vi "MPS_main.vi"() -> ()   [LabVIEW 2021] (continued)
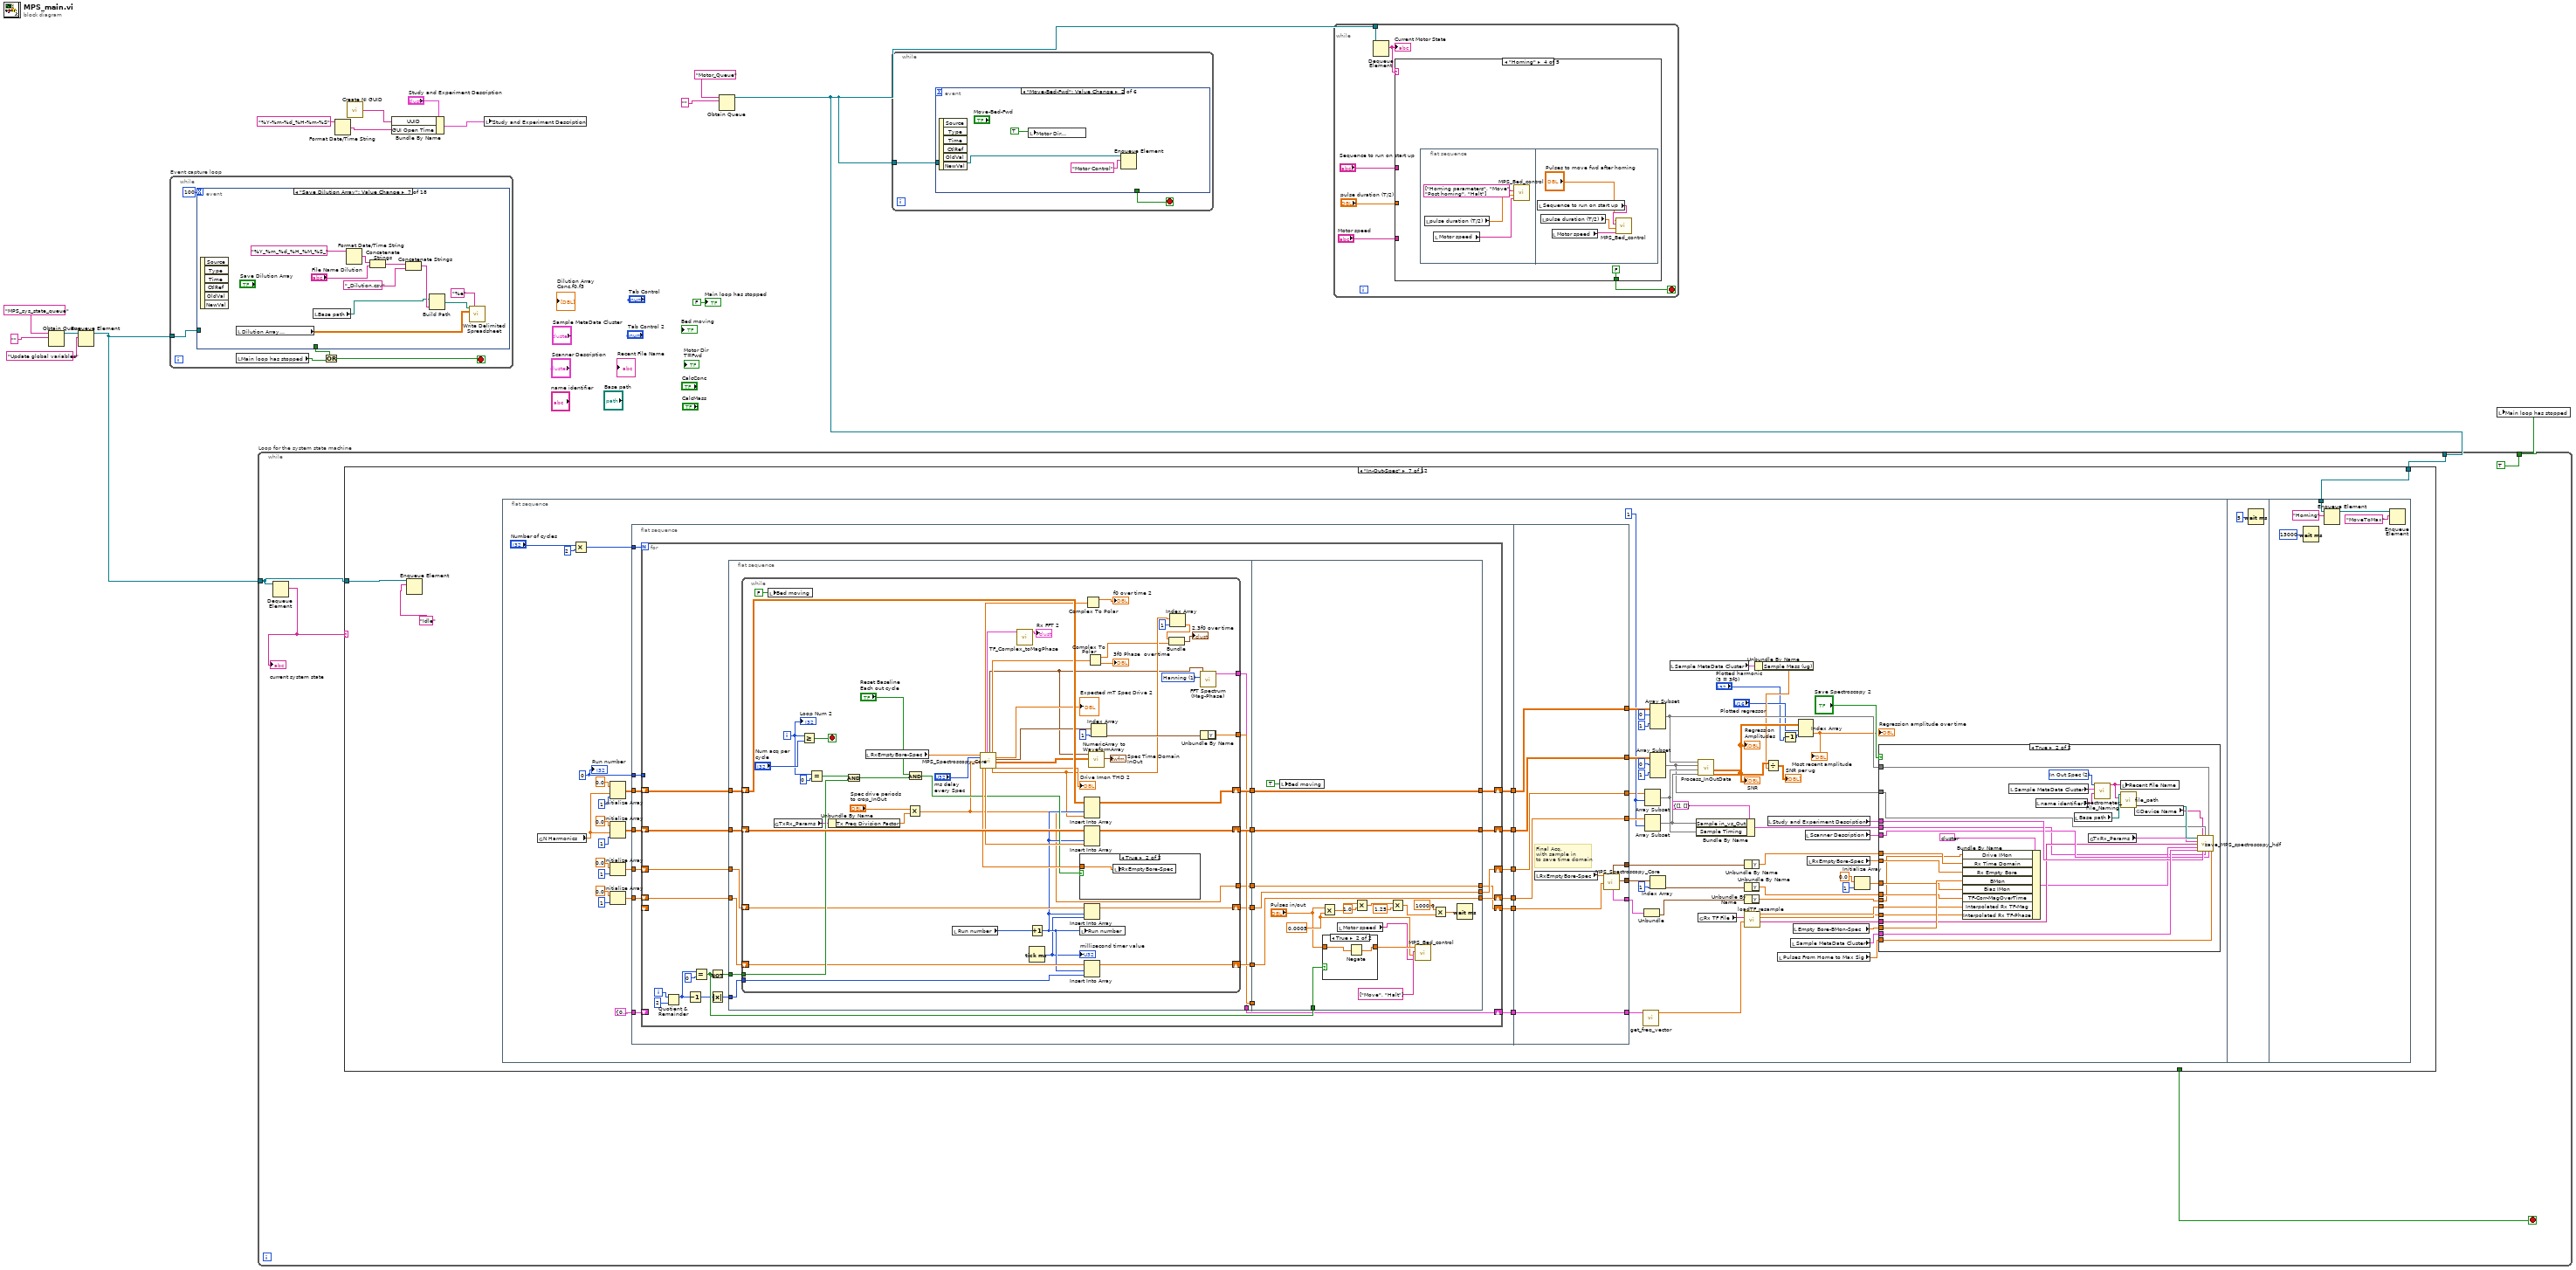
[diagram p0: block diagram]
diagram:
  n1 = Obtain Queue(name (unnamed)="MPS_sys_state_queue", element data type="") -> (queue out=w11:refnum<queue>)  [unwired: 3 in, 2 out]
  n2 = Enqueue Element(queue=w11, element="Update global variables") -> (queue out=w9:refnum<queue>)  [unwired: 2 in, 2 out]
  n3 = while "Event capture loop" {
    tunnel: w9 -> [w19]
    stop <- w16 stop-if-true
    n4 = event shown="[6] \"Save Dilution Array\": Value Change" {
      selector: _ -> [_ _ _ _ _ _ _ _ _ _ _ _ _ _ _ _ _ _]
      dyn-events: _ -> [_ _ _ _ _ _ _ _ _ _ _ _ _ _ _ _ _ _]
      timeout: 100 -> [_ _ _ _ _ _ _ _ _ _ _ _ _ _ _ _ _ _]
      tunnel: w19 -> [_ w22 _ w31 w33 _ _ _ w74 w78 w80 w82 w84 _ _ _ w105 w108]
      tunnel: [FALSE ("x") _ _ _ _ _ _ _ _ _ _ _ _ _ _ _ _ TRUE ("x")] -> w17
      event Timeout {
        n5 = event-data() -> ()  [unwired: 1 in, 3 out]
      }
      event "Run Sys Ref Meas": Value Change {
        n6 = event-data() -> ()  [unwired: 1 in, 6 out]
        n7 = Enqueue Element(queue=w22, element="System Reference Measurement") -> ()  [unwired: 2 in, 3 out]
      }
      event "Divide Mass by X": Value Change {
        n8 = event-data() -> ()  [unwired: 1 in, 6 out]
        n9 = local read "Sample MetaData Cluster"() -> (w29:T1)
        n10 = Unbundle By Name(w29) -> ("Sample Mass (ug)"=w30:dbl, "Sample Conc(mg/mL)"=w26:dbl)
        n11 = Divide(x=w30, y="Divide By val") -> (x/y=w27:dbl)
        n12 = Divide(x=w26, y="Divide By val") -> (x/y=w24:dbl)
        n13 = Bundle By Name(cluster=w29, "Sample Mass (ug)"=w27, "Sample Conc(mg/mL)"=w24) -> (w28:T1)
        n14 = local write "Sample MetaData Cluster"(w28) -> ()
      }
      event "Run Spectroscopy": Value Change {
        n15 = event-data() -> ()  [unwired: 1 in, 6 out]
        n16 = Enqueue Element(queue=w31, element="Spectroscopy") -> ()  [unwired: 2 in, 3 out]
      }
      event "Run DilutionAdd": Value Change {
        n17 = event-data() -> ()  [unwired: 1 in, 6 out]
        n18 = Enqueue Element(queue=w33, element="Acquire Dilution Data") -> ()  [unwired: 2 in, 3 out]
      }
      event "Clear Dilution Array": Value Change {
        n19 = event-data() -> ()  [unwired: 1 in, 6 out]
        n20 = Initialize Array(0.0 ("element"), 0 ("dimension size"), 3 ("dimension size")) -> (w35:dbl[][])
        n21 = local write "Dilution Array\nConc,f0,f3"(w35) -> ()
        n22 = Index Array(array=w35, index (col)=0 ("disabled index (col)")) -> (element=w42:dbl[])  [unwired: 1 in]
        n23 = Index Array(array=w35, index (col)=2 ("disabled index (col)")) -> (element=w43:dbl[])  [unwired: 1 in]
        n24 = call <vilib>:"Linear Fit.vi"("Y"=w43, "X"=w42) -> ("Best Linear Fit"=w41:dbl[])  [unwired: 9 in, 4 out]
        n25 = Bundle(w42, w43) -> (w39:cluster{dbl[], dbl[]})  [unwired: 1 in]
        n26 = call <vilib>:"Correlation Coefficient (Spearman).vi"("Y"=w43, "X"=w42) -> ()  [unwired: 8 in, 2 out]
        n27 = Bundle(w42, "Best Linear Fit"=w41) -> (w40:cluster{dbl[], "Best Linear Fit":dbl[]})  [unwired: 1 in]
        n28 = Build Array(w40, w39) -> (w38:cluster{dbl[], "Best Linear Fit":dbl[]}[])
        n29 = local write "3f0 vs Mass"(w38) -> ()
      }
      event "Save Dilution Array": Value Change {
        n30 = event-data() -> ()  [unwired: 1 in, 6 out]
        n31 = local read "Dilution Array\nConc,f0,f3"() -> (w49:dbl[][])
        n32 = local read "Base path"() -> (w47:path)
        n33 = Format Date/Time String(time format string (%c)="%Y_%m_%d_%H_%M_%S_") -> (date/time string=w54:string)  [unwired: 2 in]
        n34 = Concatenate Strings(w54, "File Name Dilution") -> (w56:string)
        n35 = Concatenate Strings(w56, "_Dilution.csv" ("string")) -> (w55:string)
        n36 = Build Path(base path=w47, name or relative path=w55) -> (appended path=w50:path)
        n37 = call-poly <vilib>:"Write Delimited Spreadsheet.vi"("file path (dialog if empty)"=w50, "format (%.3f)"="%e", "2D data"=w49) -> ()  [unwired: 11 in, 2 out]
      }
      event "Delete Last Meas": Value Change {
        n38 = event-data() -> ()  [unwired: 1 in, 6 out]
        n39 = local read "Dilution Array\nConc,f0,f3"() -> (w72:dbl[][])
        n40 = Array Size(array=w72) -> (size(s)=w71:i32[])
        n41 = Index Array(array=w71, index=0) -> (element=w69:i32)
        n42 = Decrement(x=w69) -> (x-1=w68:i32)
        n43 = Array Subset(array=w72, index (row)=0 ("index"), length (row)=w68, index (col)=0 ("index")) -> (w58:dbl[][])  [unwired: 1 in]
        n44 = local write "Dilution Array\nConc,f0,f3"(w58) -> ()
        n45 = Index Array(array=w58, index (col)=0 ("disabled index (col)")) -> (element=w64:dbl[])  [unwired: 1 in]
        n46 = Index Array(array=w58, index (col)=2 ("disabled index (col)")) -> (element=w65:dbl[])  [unwired: 1 in]
        n47 = call <vilib>:"Linear Fit.vi"("Y"=w65, "X"=w64) -> ("Best Linear Fit"=w63:dbl[])  [unwired: 9 in, 4 out]
        n48 = Bundle(w64, w65) -> (w61:cluster{dbl[], dbl[]})  [unwired: 1 in]
        n49 = call <vilib>:"Correlation Coefficient (Spearman).vi"("Y"=w65, "X"=w64) -> ()  [unwired: 8 in, 2 out]
        n50 = Bundle(w64, "Best Linear Fit"=w63) -> (w62:cluster{dbl[], "Best Linear Fit":dbl[]})  [unwired: 1 in]
        n51 = Build Array(w62, w61) -> (w57:cluster{dbl[], "Best Linear Fit":dbl[]}[])
        n52 = local write "3f0 vs Mass"(w57) -> ()
      }
      event "Run in-out spec": Value Change {
        n53 = event-data() -> ()  [unwired: 1 in, 6 out]
        n54 = for {
          N: "Number of \nsaved runs" -> [_]
          tunnel: w74 -> [w75]
          n55 = flat-sequence {
            tunnel: w75 -> [w76]
            frame #0 {
              n56 = Enqueue Element(queue=w76, element="In-Out-Spec") -> ()  [unwired: 2 in, 3 out]
            }
            frame #1 {
            }
          }
        }
      }
      event "Run Mag": Value Change {
        n57 = event-data() -> ()  [unwired: 1 in, 6 out]
        n58 = Enqueue Element(queue=w78, element="Magnetometry") -> ()  [unwired: 2 in, 3 out]
      }
      event "Acq Baseline": Value Change {
        n59 = event-data() -> ()  [unwired: 1 in, 6 out]
        n60 = Enqueue Element(queue=w80, element="Acquire Empty Bore") -> ()  [unwired: 2 in, 3 out]
      }
      event "Zero Baseline": Value Change {
        n61 = event-data() -> ()  [unwired: 1 in, 6 out]
        n62 = Enqueue Element(queue=w82, element="Zero Baseline") -> ()  [unwired: 2 in, 3 out]
      }
      event "Run Cal BMon": Value Change {
        n63 = event-data() -> ()  [unwired: 1 in, 6 out]
        n64 = Enqueue Element(queue=w84, element="Cal_BMon") -> ()  [unwired: 2 in, 3 out]
      }
      event "CalcMass": Value Change {
        n65 = event-data() -> ()  [unwired: 1 in, 6 out]
        n66 = local read "Sample MetaData Cluster"() -> (w90:T1)
        n67 = Unbundle By Name(w90) -> ("Sample Volume (uL)"=w89:dbl, "Sample Conc(mg/mL)"=w88:dbl)
        n68 = Multiply(x=w89, y=w88) -> (x*y=w86:dbl)
        n69 = Bundle By Name(cluster=w90, "Sample Mass (ug)"=w86) -> (w87:T1)
        n70 = local write "Sample MetaData Cluster"(w87) -> ()
      }
      event "CalcConc": Value Change {
        n71 = event-data() -> ()  [unwired: 1 in, 6 out]
        n72 = local read "Sample MetaData Cluster"() -> (w95:T1)
        n73 = Unbundle By Name(w95) -> ("Sample Mass (ug)"=w94:dbl, "Sample Volume (uL)"=w93:dbl)
        n74 = Divide(x=w94, y=w93) -> (x/y=w91:dbl)
        n75 = Bundle By Name(cluster=w95, "Sample Conc(mg/mL)"=w91) -> (w92:T1)
        n76 = local write "Sample MetaData Cluster"(w92) -> ()
      }
      event "Toggle fan": Value Change {
        n77 = event-data() -> ()  [unwired: 1 in, 6 out]
        n78 = global read "MPS_global_variables.vi" "Fan Control Line"() -> (w100:tag)
        n79 = call-poly <vilib>:"DAQmx Create Virtual Channel.vi"("lines"=w100) -> ("task out"=w102:refnum<k21>, "error out"=w103:errorcluster)  [unwired: 13 in]
        n80 = call-poly <vilib>:"DAQmx Write.vi"("task/channels in"=w102, "data"="Toggle fan", "error in"=w103) -> ("task out"=w99:refnum<k21>, "error out"=w98:errorcluster)  [unwired: 10 in, 1 out]
        n81 = call <vilib>:"DAQmx Stop Task.vi"("task/channels in"=w99, "error in"=w98) -> ("task out"=w97:refnum<k21>, "error out"=w96:errorcluster)  [unwired: 12 in]
        n82 = call <vilib>:"DAQmx Clear Task.vi"("task in"=w97, "error in"=w96) -> ()  [unwired: 13 in, 1 out]
      }
      event "Update global variables Button": Value Change {
        n83 = event-data() -> ()  [unwired: 1 in, 6 out]
        n84 = Enqueue Element(queue=w105, element="Update global variables") -> ()  [unwired: 2 in, 3 out]
      }
      event "stop": Value Change {
        n85 = event-data() -> ()  [unwired: 1 in, 6 out]
        n86 = Enqueue Element(queue=w108, element="Halt") -> ()  [unwired: 2 in, 3 out]
      }
    }
    n87 = local read "Main loop has stopped"() -> (w18:bool)
    n88 = Or(x=w17, y=w18) -> (x .or. y?=w16:bool)
  }
  n89 = Format Date/Time String(time format string (%c)="%Y-%m-%d_%H-%m-%S") -> (date/time string=w4:string)  [unwired: 2 in]
  n90 = call <vilib>:"Create NI GUID.vi"() -> ("NI GUID"=w7:string)
  n91 = Bundle By Name(cluster="Study and Experiment Description", "UUID"=w7, "GUI Open Time"=w4) -> (w6:T5)
  n92 = local write "Study and Experiment Description"(w6) -> ()
  n93 = Obtain Queue(name (unnamed)="Motor_Queue", element data type="") -> (queue out=w1:refnum<queue>)  [unwired: 3 in, 2 out]
  n94 = while "Loop for the system state machine" {
    tunnel: w9 -> [w111]
    tunnel: [TRUE ("Main loop has stopped")] -> w12
    tunnel: w1 -> [w109]
    stop <- w113 stop-if-true
    n95 = Dequeue Element(queue=w111) -> (element=w110:string)  [unwired: 2 in, 3 out]
    "current system state" <- w110
    n96 = case shown="\"In-Out-Spec\"" w110 {
      tunnel: [_ _ _ _ _ _ _ _ _ _ _ TRUE] -> w113
      tunnel: w111 -> [_ w116 w187 w335 w388 w532 w546 _ w820 w917 w981 _]
      tunnel: w109 -> [_ _ _ _ _ _ w545 _ _ _ _ _]
      frame "Idle", Default {
      }
      frame "Update global variables" {
        n97 = Enqueue Element(queue=w116, element="Idle") -> ()  [unwired: 2 in, 3 out]
        n98 = flat-sequence {
          tunnel: [w124] -> w114
          tunnel: w114 -> [w132]
          frame #0 {
            n99 = Unbundle By Name("TxRx_Params") -> ("sample rate"=w128:dbl, "Tx Freq Division Factor"=w126:dbl, "Drive Periods per Bias"=w125:dbl)
            n100 = global read "MPS_global_variables.vi" "N Harmonics"() -> (w120:dbl)
            n101 = Subtract(x=w120, y=2.0) -> (x-y=w121:dbl)
            n102 = Divide(x=w128, y=w126) -> (x/y=w123:dbl)
            n103 = for {
              N: w121 -> [_]
              tunnel: [w130] -> w118 mode=indexing
              i -> [w131]
              n104 = Add(x=w131, y=2) -> (x+y=w130:i32)
            }
            n105 = Divide(x=w123, y=w125) -> (x/y=w127:dbl)
            n106 = Multiply(x=w123, y=w118) -> (x*y=w117:dbl[])
            n107 = Bundle By Name(cluster="TxRx_Params", "Tx freq"=w123, "Bias freq"=w127, "TX harmonics"=w117) -> (w124:T2)
            n108 = global write "MPS_global_variables.vi" "TxRx_Params"(w124) -> ()
          }
          frame #1 {
            n109 = local write "TxRx_Params"(w132) -> ()
          }
        }
      }
      frame "System Reference Measurement" {
        w146 = dbl[][] [] ("array")
        n110 = Enqueue Element(queue=w187, element="Idle") -> ()  [unwired: 2 in, 3 out]
        n111 = global read "MPS_global_variables.vi" "N Harmonics"() -> (w133:dbl)
        n112 = Initialize Array(0.0 ("element"), w133, 0 ("dimension size")) -> (w184:dbl[][])
        n113 = Initialize Array(0.0 ("element"), w133, 0 ("dimension size")) -> (w181:dbl[][])
        n114 = for {
          N: "Num Avgs SRM" -> [_]
          tunnel: "Num Avgs SRM" -> [_]
          shift-right: [w254] -> w151
          shift-left: w184 -> [w284]
          shift-right: [w253] -> w160
          shift-left: w181 -> [w283]
          shift-right: [w273] -> _
          shift-left: w146 -> [w280]
          shift-right: [w272] -> _
          shift-left: w146 -> [w277]
          shift-right: [w247] -> _
          shift-left: w146 -> [w274]
          shift-right: [w261] -> _
          shift-left: w146 -> [w271]
          shift-right: [w263] -> _
          shift-left: w146 -> [w270]
          shift-right: [w232] -> w145
          shift-left: _ -> [_]
          tunnel: [w228] -> w136
          i -> [w282]
          # "Rx FFT"
          # "PSD"
          # "Tx FFT"
          n115 = global read "MPS_global_variables.vi" "TxRx_Params"() -> (w289:T2)
          n116 = global read "MPS_global_variables.vi" "TxRx_Params"() -> (w255:T2)
          n117 = local read "RxEmptyBore-Spec"() -> (w291:dbl[])
          n118 = Unbundle By Name(w289) -> ("Tx Freq Division Factor"=w288:dbl)
          n119 = Multiply(x="Spec Tx periods\nto crop SRM", y=w288) -> (x*y=w227:dbl)
          n120 = Unbundle By Name(w255) -> ("TX harmonics"=w242:dbl[], "Tx freq"=w240:dbl)
          n121 = call "MPS_Spectroscopy_Core.vi"("EmptyBoreBaseline_Spec"=w291, "ms delay"="ms delay SRM", "Spec samples\nto crop"=w227) -> ("phase f1-f9"=w281:dbl[], "TF Corr Rx FFT complex"=w279:T12, "TF units from loaded file"=w228:string, "TxIMon cluster"=w222:T13, "mag f1-f9"=w285:dbl[])  [unwired: 2 in, 10 out]
          n122 = Unbundle(w222) -> ("TF Corr Rx FFT complex"=w221:T12)  [unwired: 1 out]
          n123 = call "TF_Complex_toMagPhase.vi"("TF Corr Rx FFT Mag"=w221) -> ("phase"=w268:dbl[], "magnitude"=w269:dbl[])  [unwired: 4 in, 5 out]
          n124 = call "TF_Complex_toMagPhase.vi"("TF Corr Rx FFT Mag"=w279) -> ("phase"=w276:dbl[], "magnitude"=w278:dbl[], "Freq array"=w220:dbl[], "PSD"=w275:dbl[])  [unwired: 4 in, 3 out]
          n125 = Equal?(x=0, y=w282) -> ()  [unwired: 1 out]
          n126 = Insert Into Array(array=w274, new element=w275) -> (w247:dbl[][])  [unwired: 2 in]
          n127 = Insert Into Array(array=w277, new element=w276) -> (w272:dbl[][])  [unwired: 2 in]
          n128 = Insert Into Array(array=w271, new element=w269) -> (w261:dbl[][])  [unwired: 2 in]
          n129 = Insert Into Array(array=w270, new element=w268) -> (w263:dbl[][])  [unwired: 2 in]
          n130 = Insert Into Array(array=w280, new element=w278) -> (w273:dbl[][])  [unwired: 2 in]
          n131 = Insert Into Array(array=w284, index (col)=w282, new element=w285) -> (w254:dbl[][])  [unwired: 1 in]
          n132 = Insert Into Array(array=w283, index (col)=w282, new element=w281) -> (w253:dbl[][])  [unwired: 1 in]
          n133 = Insert Into Array(array=w242, index=0, new element=w240) -> (w239:dbl[])
          n134 = Polar To Complex(1:w263, 2:w261) -> (0:w262:cdb[][])
          n135 = Polar To Complex(1:w272, 2:w273) -> (0:w267:cdb[][])
          n136 = Polar To Complex(1:w253, 2:w254) -> (0:w245:cdb[][])
          n137 = Transpose 2D Array(2D array=w262) -> (transposed array=w264:cdb[][])
          n138 = Transpose 2D Array(2D array=w267) -> (transposed array=w266:cdb[][])
          n139 = Transpose 2D Array(2D array=w247) -> (transposed array=w265:dbl[][])
          n140 = for {
            tunnel: w245 -> [w295] mode=indexing
            tunnel: [w294] -> w244 mode=indexing
            tunnel: [w292] -> w243 mode=indexing
            n141 = call "mean_std_var_Complex.vi"("Input Array"=w295) -> ("standard deviation"=w294:dbl, "mean"=w293:cdb)  [unwired: 8 in, 1 out]
            n142 = Complex To Polar(r * e^(i*theta)=w293) -> (r=w292:dbl)  [unwired: 1 out]
          }
          n143 = for {
            tunnel: w265 -> [w302] mode=indexing
            tunnel: [w304] -> w231 mode=indexing
            tunnel: [w303] -> w230 mode=indexing
            tunnel: w266 -> [w301] mode=indexing
            tunnel: [w300] -> w238 mode=indexing
            tunnel: [w299] -> w229 mode=indexing
            tunnel: w264 -> [w298] mode=indexing
            tunnel: [w297] -> w237 mode=indexing
            tunnel: [w296] -> w233 mode=indexing
            n144 = call "mean_std_var_Complex.vi"("Input Array"=w301) -> ("standard deviation"=w299:dbl, "mean"=w300:cdb)  [unwired: 8 in, 1 out]
            n145 = call "mean_std_var_Complex.vi"("Input Array"=w302) -> ("standard deviation"=w303:dbl, "mean"=w304:cdb)  [unwired: 8 in, 1 out]
            n146 = call "mean_std_var_Complex.vi"("Input Array"=w298) -> ("standard deviation"=w296:dbl, "mean"=w297:cdb)  [unwired: 8 in, 1 out]
          }
          n147 = Bundle("Freq array"=w220, w229) -> (w251:cluster{"Freq array":dbl[], dbl[]})  [unwired: 1 in]
          n148 = Bundle("Freq array"=w220, w230) -> (w250:cluster{"Freq array":dbl[], dbl[]})  [unwired: 1 in]
          n149 = Bundle("TX harmonics"=w239, w243) -> (w258:cluster{"TX harmonics":dbl[], dbl[]})  [unwired: 1 in]
          n150 = Bundle("Freq array"=w220, w231) -> (w260:cluster{"Freq array":dbl[], cdb[]})  [unwired: 1 in]
          n151 = Complex To Polar(r * e^(i*theta)=w237) -> (r=w226:dbl[], theta=w234:dbl[])
          n152 = Complex To Polar(r * e^(i*theta)=w238) -> (r=w236:dbl[], theta=w235:dbl[])
          n153 = Bundle("Freq array"=w220, w236) -> (w259:cluster{"Freq array":dbl[], dbl[]})  [unwired: 1 in]
          n154 = Bundle("TX harmonics"=w239, w244) -> (w252:cluster{"TX harmonics":dbl[], dbl[]})  [unwired: 1 in]
          n155 = Build Array(w258, w259, w260) -> (→"mean(FFT) mag":cluster{"Freq array":dbl[], cdb[]}[])
          n156 = Build Array(w252, w251, w250) -> (→"std(FFT)":cluster{"Freq array":dbl[], dbl[]}[])
          n157 = Bundle By Name(cluster=w221, "magnitude"=w226) -> (w225:T12)
          n158 = Bundle("Freq array"=w220, w226) -> (→"mean(FFT) Tx Current":cluster{"Freq array":dbl[], dbl[]})  [unwired: 1 in]
          n159 = Bundle("Freq array"=w220, w233) -> (→"std(FFT)  Tx Current":cluster{"Freq array":dbl[], dbl[]})  [unwired: 1 in]
          n160 = Bundle(w236, w235, w229, w231, w230, w226, w234, w233, "Freq array"=w220) -> (w232:T14)  [unwired: 1 in]
          n161 = Array Size(array=w233) -> (size(s)=→"size(s)":i32)
          n162 = call "FFT-THD.vi"("TF Corr IMon FFT"=w225) -> ("THD"=w224:dbl)  [unwired: 10 in]
          "Mean_IMon_THD" <- w224
          n163 = expression code="20*log(x)"(w224) -> (→"MeanIMonTHD_dB":dbl)
          "Loop Num 3" <- w282
        }
        n164 = Polar To Complex(1:w160, 2:w151) -> (0:w167:cdb[][])
        n165 = Array Subset(array=w151, index (row)=2 ("index"), length (row)=1 ("length"), index (col)=0 ("index")) -> (w158:dbl[][])  [unwired: 1 in]
        n166 = case shown="False" "Apply drift \ncorrection?" {
          tunnel: w167 -> [w189 w191]
          tunnel: [w189 w190] -> w166
          frame False {
          }
          frame True {
            n167 = call "RemoveDrift.vi"("Drift degree"=3.0, "Data In"=w191) -> ("Data Drift Removed"=w190:cdb[][])  [unwired: 9 in]
          }
        }
        n168 = Reshape Array(w158, "Num Avgs SRM") -> (w156:dbl[])
        n169 = Complex To Polar(r * e^(i*theta)=w166) -> (r=w149:dbl[][], theta=w148:dbl[][])
        n170 = Initialize Array(0.0 ("element"), w133) -> (w178:dbl[])
        n171 = Initialize Array(0.0 ("element"), w133) -> (w177:dbl[])
        n172 = Initialize Array(0.0 ("element"), w133) -> (w174:dbl[])
        n173 = Initialize Array(0.0 ("element"), w133) -> (w173:dbl[])
        n174 = Array Subset(array=w149, index (row)=2 ("index"), length (row)=1 ("length"), index (col)=0 ("index")) -> (w157:dbl[][])  [unwired: 1 in]
        n175 = Reshape Array(w157, "Num Avgs SRM") -> (w155:dbl[])
        n176 = for {
          tunnel: w149 -> [w219] mode=indexing
          tunnel: w148 -> [w218] mode=indexing
          shift-right: [w214] -> w134
          shift-left: w178 -> [w217]
          shift-right: [w215] -> w170
          shift-left: w177 -> [w216]
          shift-right: [w208] -> w169
          shift-left: w174 -> [w211]
          shift-right: [w209] -> w168
          shift-left: w173 -> [w210]
          i -> [w207]
          n177 = call <vilib>:"Std Deviation and Variance.vi"("X"=w219) -> ("mean"=w213:dbl, "standard deviation"=w206:dbl)  [unwired: 1 in, 1 out]
          n178 = call <vilib>:"Std Deviation and Variance.vi"("X"=w218) -> ("mean"=w212:dbl, "standard deviation"=w205:dbl)  [unwired: 1 in, 1 out]
          n179 = Replace Array Subset(array=w217, new element=w213, index=w207) -> (w214:dbl[])
          n180 = Replace Array Subset(array=w216, new element=w212, index=w207) -> (w215:dbl[])
          n181 = Replace Array Subset(array=w211, new element=w206, index=w207) -> (w208:dbl[])
          n182 = Replace Array Subset(array=w210, new element=w205, index=w207) -> (w209:dbl[])
        }
        "Std of mags TF Corr" <- w169
        "Mean of mags TF Corr" <- w134
        n183 = Build Array(w156, w155) -> (→"Waveform Graph":dbl[][])
        n184 = Unbundle(w145) -> (w144:dbl[], w143:dbl[], w142:dbl[], w141:cdb[], w140:dbl[], w139:dbl[], w138:dbl[], w137:dbl[], "Freq array"=w135:dbl[])
        n185 = Bundle By Name(cluster=T7 {"Mean of Mags\nTF Corrected"=[0.11891545467140323, 3.2359956159889795e-06, 4.683456836791031e-06, 2.2974949759077933e-06, 7.335205151756684e-06, 2.2780944083652307e-06, 3.6882771584744806e-06, 3.943947428053956e-06, 5.677081505502577e-06], "Mean of Phase\nTF Corrected"=[1.2189052024941316, 1.3335507267391822, 1.0623290638021972, 1.2312410772168787, -2.3901914592329807, -0.9400489906160769, -0.38268681350318423, -1.5651667523229502, 2.0808572423614278], "Std of Mags\nTF Corrected"=[1.7822550794636106e-06, 1.362064067189915e-06, 1.4384290038051052e-06, 1.2224491171904712e-06, 1.5415851022050893e-06, 1.1506615886407483e-06, 1.5896649122010608e-06, 1.392010277859625e-06, 1.977168509459674e-06], "Std of Phase\nTF Corrected 4"=[0.00044396269347641464, 2.1812626503429993, 0.36980551924146593, 1.6282356086497982, 1.5207696449300456, 1.7213228694360245, 2.6615550793626337, 0.5214361017901513, 1.6763493877670135], "All Mag"=[], "All Phase"=[], "RxFFTMag_AllFreqs"=[], "RxFFTPhase_AllFreqs"=[], "Std-RxFFT_AllFreqs"=[], "Rx_PSD_AllFreqs"=[], "Std-Rx_PSD_AllFreqs"=[], "TxFFTMag_AllFreqs"=[], "TxFFTPhase_AllFreqs"=[], "Std-TxFFT_AllFreqs"=[], "freqs"=[]} ("SRM Stats"), "Mean of Mags\nTF Corrected"=w134, "Mean of Phase\nTF Corrected"=w170, "Std of Mags\nTF Corrected"=w169, "Std of Phase\nTF Corrected 4"=w168, "All Mag"=w149, "All Phase"=w148, "RxFFTMag_AllFreqs"=w144, "RxFFTPhase_AllFreqs"=w143, "Std-RxFFT_AllFreqs"=w142, "Rx_PSD_AllFreqs"=w141, "Std-Rx_PSD_AllFreqs"=w140, "TxFFTMag_AllFreqs"=w139, "TxFFTPhase_AllFreqs"=w138, "Std-TxFFT_AllFreqs"=w137, "freqs"=w135) -> (w152:T7)
        n186 = local read "Pulses From Home to Max Sig"() -> (w172:dbl)
        n187 = case shown="True" "Save SRM" {
          tunnel: w172 -> [_ w201]
          tunnel: w152 -> [_ w194]
          tunnel: w136 -> [_ w193]
          frame False {
          }
          frame True {
            w195 = u16 3 items=["Spec.", "Mag.", "In Out Spec", "SRM", "", ""] ("Ring")
            n188 = local read "name identifier"() -> (w197:string)
            n189 = local read "Scanner Description"() -> (w200:T4)
            n190 = local read "Study and Experiment Description"() -> (w199:T5)
            n191 = local read "Base path"() -> (w198:path)
            n192 = call "Spectrometer_File_Naming.vi"("Description"=w197, "Ring"=w195) -> ("Output Name"=w196:string)  [unwired: 9 in]
            n193 = call "file_path.vi"("name identifier"=w196, "Base path"=w198) -> ("HDF path"=w203:path)  [unwired: 7 in, 2 out]
            n194 = global read "MPS_global_variables.vi" "TxRx_Params"() -> (w202:T2)
            n195 = local write "Recent File Name"(w196) -> ()
            n196 = call "save_MPS_SystemRef_hdf.vi"("file path"=w203, "Device Name"=tag "H1", "TxRx_Params"=w202, "Rx_f0-f8 Units"=w193, "SRM Stats"=w194, "Study and Experiment Description"=w199, "Scanner Description"=w200, "Points from home to max"=w201) -> ()  [unwired: 8 in]
          }
        }
      }
      frame "Cal_BMon" {
        w315 = T15 1 items=["Rectangle"=0, "Hanning"=1, "Hamming"=2, "Blackman-Harris"=3, "Exact Blackman"=4, "Blackman"=5, "Flat Top"=6, "4 Term B-Harris "=7, "7 Term B-Harris"=8, "Low Sidelobe"=9, "Blackman Nuttall"=11, "Triangle"=30, "Bartlett-Hanning"=31, "Bohman"=32, "Parzen"=33, "Welch"=34, "Kaiser"=60, "Dolph-Chebyshev"=61, "Gaussian"=62] ("window")
        w321 = waveform(dbl) {"t0"=timestamp(0 s since 1904-01-01), "dt"=1.0, "Y"=[]} ("Waveform")
        # "Data queue"
        n197 = Enqueue Element(queue=w335, element="Idle") -> ()  [unwired: 2 in, 3 out]
        n198 = global read "MPS_global_variables.vi" "TxRx_Params"() -> (w328:T2)
        n199 = Obtain Queue(element data type=w321) -> (queue out=w337:refnum<queue>)  [unwired: 4 in, 2 out]
        n200 = global read "MPS_global_variables.vi" "TxRx_Params"() -> (w312:T2)
        n201 = Unbundle By Name(w328) -> ("Tx cycles\nSpectroscopy"=w324:dbl, "sample rate"=w327:dbl, "Tx freq"=w326:dbl)
        n202 = Obtain Queue(element data type=w321) -> (queue out=w336:refnum<queue>)  [unwired: 4 in, 2 out]
        n203 = call <extravilib>:"Write.vi"("element"=1 ("number of readouts")) -> ("channel"=w338:T16)  [unwired: 1 out]
        n204 = local read "Spec Tx periods\nto crop"() -> (w310:dbl)
        n205 = Unbundle By Name(w312) -> ("Tx Freq Division Factor"=w311:dbl)
        n206 = flat-sequence {
          tunnel: w337 -> [w344]
          tunnel: [w347] -> w341
          tunnel: w338 -> [w348]
          tunnel: w336 -> [w347]
          tunnel: w322 -> [w345]
          tunnel: [w342] -> w314
          tunnel: w341 -> [w351]
          tunnel: w338 -> [w354]
          tunnel: w322 -> [w352]
          tunnel: [w349] -> w320
          frame #0 {
            n207 = Dequeue Element(queue=w344) -> (element=w342:waveform(dbl))  [unwired: 2 in, 3 out]
            n208 = call "MPS_transmit_receive.vi"("samples per readout"=w345, "Use Bias?"=FALSE, "InputChans"=enum16{"Rx", "BiasIMon", "TxIMon", "BMon"}."TxIMon", "channel input for max readouts"=w348, "Measurement Queue"=w344) -> ()  [unwired: 7 in]
          }
          frame #1 {
            n209 = Dequeue Element(queue=w351) -> (element=w349:waveform(dbl))  [unwired: 2 in, 3 out]
            n210 = call "MPS_transmit_receive.vi"("samples per readout"=w352, "Use Bias?"=FALSE, "InputChans"=enum16{"Rx", "BiasIMon", "TxIMon", "BMon"}."BMon", "channel input for max readouts"=w354, "Measurement Queue"=w351) -> ()  [unwired: 7 in]
          }
        }
        n211 = Divide(x=w327, y=w326) -> (x/y=w325:dbl)
        n212 = Multiply(x=w324, y=w325) -> (x*y=w323:dbl)
        n213 = Round To Nearest(number=w323) -> (nearest integer value=w322:dbl)
        "Samples Per Acquisition" <- w322
        n214 = Multiply(x=w310, y=w311) -> (x*y=w309:dbl)
        n215 = call "Waveform_Indexing.vi"("index"=w309, "waveform"=w314) -> ("output waveform"=w313:waveform(dbl))  [unwired: 7 in]
        n216 = global read "MPS_global_variables.vi" "TxRx_Params"() -> (w331:T2)
        n217 = Unbundle By Name(w331) -> ("Tx freq"=w330:dbl)
        n218 = Bundle By Name(cluster=T8 {"sample rate"=1000000.0, "Transmit frequency"=25000.0, "Transmit amplitude"=1.577, "sample rate digital out"=40000.0, "TX cycles"=600, "sample rate DAQ1"=1000000.0, "Receive frequency"=75000.0, "Receive range"=1.0, "TX harmonics"=[50000.0, 75000.0, 100000.0, 125000.0, 150000.0, 175000.0, 200000.0, 225000.0]} ("TxRxParams"), "Transmit frequency"=w330, "Receive frequency"=w330) -> (w329:T8)
        n219 = call "Time domain Tx-TF Correction.vi"("window"=w315, "Tx Waveform"=w313) -> ("TF Corr Rx FFT complex"=w318:T12)  [unwired: 4 in, 5 out]
        n220 = call "TF_Complex_toMagPhase.vi"("TF Corr Rx FFT Mag"=w318) -> ("TF Phase"=w316:cluster{"f0":dbl, "df":dbl, "magnitude":dbl[]}, "TF Mag"=w317:cluster{"f0":dbl, "df":dbl, "magnitude":dbl[]})  [unwired: 4 in, 5 out]
        n221 = call-poly <vilib>:"FFT Spectrum (Mag-Phase).vi"("time signal"=w320) -> ("phase"=w333:cluster{"f0":dbl, "df":dbl, "phase":dbl[]}, "magnitude"=w334:cluster{"f0":dbl, "df":dbl, "magnitude":dbl[]})  [unwired: 6 in, 3 out]
        n222 = call "determine_harmonics_NHarmonics.vi"("FFT magnitude"=w317, "FFT phase"=w316, "TxRxParams"=w329) -> ("RX magnitude"=w305:dbl)  [unwired: 11 in, 5 out]
        "Meas Drive IMon Val RMS\nCal BMon" <- w305
        n223 = call "determine_harmonics_NHarmonics.vi"("FFT magnitude"=w334, "FFT phase"=w333, "TxRxParams"=w329) -> ("RX magnitude"=w306:dbl)  [unwired: 11 in, 5 out]
        "Meas BMon Val RMS" <- w306
        n224 = call "MPS_Drive_ImonScale.vi"("Drive IMon FFT Mag RMS"=w305) -> ("Amps Drive Peak"=→"Amps Drive Peak":dbl, "Expected mT Peak"=→"Expected mT peak":dbl)  [unwired: 9 in]
        n225 = Divide(x=w305, y=w306) -> (x/y=w307:dbl)
        "mT/BMon Volt" <- w307
        n226 = global write "MPS_global_variables.vi" "mT/BMon Volt"(w307) -> ()
      }
      frame "Spectroscopy" {
        n227 = Enqueue Element(queue=w388, element="Idle") -> ()  [unwired: 2 in, 3 out]
        n228 = local read "Sample MetaData Cluster"() -> (w361:T1)
        n229 = case shown="False" "Normalize to mass?" {
          frame False {
            n230 = property on="Langevin" class="XYGraph (strict)"("YScale.NameLbl.Text"="Magnetization [Am^2]" ("Y Scale.Name Label.Text")) -> ()  [unwired: 2 in, 2 out]
          }
          frame True {
            n231 = property on="Langevin" class="XYGraph (strict)"("YScale.NameLbl.Text"="Magnetization per mass [Am^2/kg]" ("Y Scale.Name Label.Text")) -> ()  [unwired: 2 in, 2 out]
          }
        }
        n232 = Unbundle By Name(w361) -> ("Sample Mass (ug)"=w360:dbl)
        n233 = Multiply(x=w360, y=1e-09) -> (x*y=w358:dbl)
        n234 = global read "MPS_global_variables.vi" "N Harmonics"() -> (w356:dbl)
        n235 = global read "MPS_global_variables.vi" "N Harmonics"() -> (w357:dbl)
        n236 = Initialize Array(0.0 ("element"), 0 ("dimension size"), w356) -> (w385:dbl[][])
        n237 = Initialize Array(0.0 ("element"), 0 ("dimension size"), w357) -> (w382:dbl[][])
        n238 = while {
          shift-right: [w482] -> w372
          shift-left: w385 -> [w483]
          tunnel: [w473] -> w381
          tunnel: [w469] -> w380
          tunnel: [w446] -> w370
          tunnel: [w459] -> w369
          tunnel: [w457] -> w368
          tunnel: [w458] -> w367
          tunnel: [w429] -> w364
          tunnel: [w427] -> w363
          tunnel: w358 -> [w423]
          shift-right: [w422] -> w355
          shift-left: w382 -> [w481]
          i -> [w450]
          stop <- w477 stop-if-true
          w470 = T15 1 items=["Rectangle"=0, "Hanning"=1, "Hamming"=2, "Blackman-Harris"=3, "Exact Blackman"=4, "Blackman"=5, "Flat Top"=6, "4 Term B-Harris "=7, "7 Term B-Harris"=8, "Low Sidelobe"=9, "Blackman Nuttall"=11, "Triangle"=30, "Bartlett-Hanning"=31, "Bohman"=32, "Parzen"=33, "Welch"=34, "Kaiser"=60, "Dolph-Chebyshev"=61, "Gaussian"=62] ("window")
          n239 = global read "MPS_global_variables.vi" "TxRx_Params"() -> (w453:T2)
          n240 = Unbundle By Name(w453) -> ("Tx Freq Division Factor"=w452:dbl)
          n241 = local read "RxEmptyBore-Spec"() -> (w476:dbl[])
          n242 = Multiply(x="Spec Tx periods\nto crop", y=w452) -> (x*y=w439:dbl)
          n243 = Equal?(x=w450, y=0) -> (x = y?=w448:bool)
          n244 = call "MPS_Spectroscopy_Core.vi"("EmptyBoreBaseline_Spec"=w476, "ms delay"="ms delay", "Spec samples\nto crop"=w439) -> ("f0 Complex"=w466:cdb, "phase f1-f9"=w474:dbl[], "TF Corr Rx FFT complex"=w444:T12, "Spec Waveform Baseline Sub"=w420:waveform(dbl), "TxIMon cluster"=w442:T13, "3f0 Complex"=w468:cdb, "mag f1-f9"=w436:dbl[], "Expected mT Spec Drive"=w471:dbl, "TF Corrected\nMagnetization over time"=w465:waveform(dbl)[], "Spec Time Domain"=w421:dbl[][], "THD"=→"THD":dbl)  [unwired: 2 in, 4 out]
          n245 = case shown="False" w448 {
            tunnel: w471 -> [w486 w500]
            tunnel: "UseFeedback" -> [w485 _]
            tunnel: "Feedback Avging" -> [w484 w498]
            frame False {
              n246 = case shown="False" w485 {
                tunnel: w486 -> [w487 w489]
                tunnel: w484 -> [_ w494]
                frame False {
                  n247 = local write "Expected mT Spec Drive"(w487) -> ()
                }
                frame True {
                  n248 = local read "Last N Drive Amp"() -> (w496:dbl[])
                  n249 = local read "Ref mT Spec Drive"() -> (w497:dbl)
                  n250 = local read "Loop Num"() -> (w495:i32)
                  n251 = call "MPS_Feedback_Spec.vi"("Ref mT"=w497, "Expected mT Spec Drive"=w489, "last N array"=w496, "Error Gain"="Error Gain", "Loop num"=w495, "Num avgs"=w494) -> ("Relative Drive"=→"Relative mT Drive":dbl, "Updated Tx Amp"=→"Updated Tx Amp":dbl, "Error"=→"Error":dbl, "Updated last N"=w493:dbl[])  [unwired: 6 in]
                  n252 = local write "Last N Drive Amp"(w493) -> ()
                  "Expected mT Spec Drive" <- w489
                }
              }
            }
            frame True {
              n253 = Initialize Array(w500, w498) -> (→"Last N Drive Amp":dbl[])
              "Ref mT Spec Drive" <- w500
            }
          }
          n254 = call "TF_Complex_toMagPhase.vi"("TF Corr Rx FFT Mag"=w444) -> ("TF Mag"=→"Rx FFT":cluster{"f0":dbl, "df":dbl, "magnitude":dbl[]})  [unwired: 4 in, 6 out]
          n255 = call "NumericArray to WaveformArray.vi"("Array input"=w421, "Ref Waveform"=w420) -> ("Array of waveforms"=→"Spec Time Domain":waveform(dbl)[])  [unwired: 9 in]
          n256 = Insert Into Array(array=w481, index (row)=w450, new element=w474) -> (w422:dbl[][])  [unwired: 1 in]
          n257 = Insert Into Array(array=w483, index (row)=w450, new element=w436) -> (w482:dbl[][])  [unwired: 1 in]
          n258 = Complex To Polar(r * e^(i*theta)=w468) -> (r=w437:dbl)  [unwired: 1 out]
          n259 = Complex To Polar(r * e^(i*theta)=w466) -> (r=→"f0 over time":dbl, theta=→"f0 Phase over time":dbl)
          n260 = Index Array(array=w465, index=1) -> (element=w463:waveform(dbl))
          n261 = Index Array(array=w436, index=1) -> (element=w434:dbl)
          n262 = Bundle(w437, w434) -> (→"3f0 over time":cluster{dbl, dbl})  [unwired: 1 in]
          n263 = Unbundle(w442) -> ("output waveform"=w441:waveform(dbl))  [unwired: 1 out]
          n264 = Unbundle By Name(w463) -> ("Y"=w446:dbl[])
          n265 = local read "Normalize to mass?"() -> (w424:bool)
          n266 = local read "Expected mT Spec Drive"() -> (w431:dbl)
          n267 = Index Array(array=w421, index (row)=2) -> (element=w432:dbl[])  [unwired: 1 in]
          n268 = local read "RxEmptyBore-Spec"() -> (w430:dbl[])
          n269 = local read "Empty Bore-BMon-Spec"() -> (w428:dbl[])
          n270 = Greater Or Equal?(x=w450, y="Max Spec Runs") -> (x >= y?=w478:bool)
          n271 = Array Subset(array=w430, index=w439) -> (w429:dbl[])  [unwired: 1 in]
          n272 = call-poly <vilib>:"FFT Spectrum (Mag-Phase).vi"("window"=w470, "time signal"=w420) -> ("magnitude"=w461:cluster{"f0":dbl, "df":dbl, "magnitude":dbl[]})  [unwired: 5 in, 4 out]
          n273 = Array Subset(array=w428, index=w439) -> (w427:dbl[])  [unwired: 1 in]
          n274 = call "PlotLangevinCore.vi"("Peak mT"=w431, "Normalize to mass?"=w424, "MassKg"=w423, "BMon"=w427, "Rx"=w432) -> ("BMon_Int_mT"=w425:dbl[], "Rx_M_t_Out"=w426:dbl[])  [unwired: 3 in, 2 out]
          n275 = call "Convert to Dynamic Data2"("Array"=w425) -> ("Dynamic Data Type"=w454:dynamicdata)  [unwired: 3 in]
          n276 = call "Convert to Dynamic Data"("Array"=w426) -> ("Dynamic Data Type"=w455:dynamicdata)  [unwired: 3 in]
          n277 = global read "MPS_global_variables.vi" "Rx TF File"() -> (w460:string)
          n278 = call "Build XY Graph"("Y Input"=w455, "X Input"=w454) -> ("XY Graph"=→"Langevin":cluster{"X":dbl[], "Y":dbl[]}[])  [unwired: 8 in, 1 out]
          n279 = call "get_freq_vector.vi"("FFT magnitude"=w461) -> ("Freq array"=w462:dbl[])  [unwired: 10 in]
          n280 = Or(x="Stop Spec", y=w478) -> (x .or. y?=w477:bool)
          n281 = Unbundle By Name(w441) -> ("Y"=w473:dbl[])
          n282 = Unbundle By Name(w420) -> ("Y"=w469:dbl[])
          n283 = call "loadTF_resample.vi"("desired freqs"=w462, "mat file name"=w460) -> ("TF units from loaded file"=w457:string, "output TF phase"=w458:dbl[], "output TF mag"=w459:dbl[])  [unwired: 7 in]
          "Loop Num" <- w450
        }
        n284 = local read "Pulses From Home to Max Sig"() -> (w366:dbl)
        n285 = Index Array(array=w372, index (col)=2 ("index")) -> (element=w379:dbl[])  [unwired: 1 in]
        n286 = Index Array(array=w372, index (col)=0 ("disabled index (col)")) -> (element=w373:dbl[])  [unwired: 1 in]
        n287 = call <vilib>:"Std Deviation and Variance.vi"("X"=w379) -> ("mean"=→"mean3f0":dbl, "standard deviation"=→"standard deviation 3f0":dbl)  [unwired: 1 in, 1 out]
        n288 = case shown="True" "Save Spectroscopy" {
          tunnel: w364 -> [_ w417]
          tunnel: w363 -> [_ w416]
          tunnel: w372 -> [_ w413]
          tunnel: w355 -> [_ w412]
          tunnel: w381 -> [_ w393]
          tunnel: w380 -> [_ w411]
          tunnel: w370 -> [_ w410]
          tunnel: w369 -> [_ w409]
          tunnel: w368 -> [_ w408]
          tunnel: w367 -> [_ w406]
          tunnel: w366 -> [_ w402]
          frame False {
          }
          frame True {
            w395 = u16 0 items=["Spec.", "Mag.", "In Out Spec"] ("Ring")
            n289 = Initialize Array(0.0 ("element"), 1 ("dimension size")) -> (w403:dbl[])
            n290 = Bundle By Name(cluster=T9 {"Drive IMon"=array[500000 elements], "Rx Time Domain"=array[500000 elements], "Rx Empty Bore"=array[500000 elements], "BMon"=array[500000 elements], "Bias IMon"=array[500000 elements], "TF-Corr-MagOverTime"=[], "Interpolated Rx TF-Mag"=[], "Interpolated Rx TF-Phase"=[]} ("Time Domain Cluster"), "Drive IMon"=w393, "Rx Time Domain"=w411, "Rx Empty Bore"=w417, "BMon"=w416, "Bias IMon"=w403, "TF-Corr-MagOverTime"=w410, "Interpolated Rx TF-Mag"=w409, "Interpolated Rx TF-Phase"=w406) -> (w418:T9)
            n291 = local read "Sample MetaData Cluster"() -> (w396:T1)
            n292 = local read "name identifier"() -> (w397:string)
            n293 = local read "Study and Experiment Description"() -> (w400:T5)
            n294 = local read "Sample MetaData Cluster"() -> (w399:T1)
            n295 = local read "Base path"() -> (w398:path)
            n296 = local read "Scanner Description"() -> (w401:T4)
            n297 = global read "MPS_global_variables.vi" "TxRx_Params"() -> (w414:T2)
            n298 = call "Spectrometer_File_Naming.vi"("Description"=w397, "Sample MetaData Cluster"=w396, "Ring"=w395) -> ("Output Name"=w394:string)  [unwired: 8 in]
            n299 = local write "Recent File Name"(w394) -> ()
            n300 = call "file_path.vi"("name identifier"=w394, "Base path"=w398) -> ("HDF path"=w415:path)  [unwired: 7 in, 2 out]